vi "HFRR ADV v043.vi"() -> ()   [LabVIEW 2025] (continued)
  }
  n1338 = while {
    tunnel: w42 -> [_]
    tunnel: w28 -> [_]
    stop <- w1527 stop-if-true
    # "New Adv Logics"
    n1339 = local read "Main Tab"() -> (w1508:T2)
    n1340 = local read "Main Tab"() -> (w1525:T2)
    n1341 = local read "Sign In"() -> (w1524:bool)
    n1342 = case shown="\"Adv Scar\"" w1508 {
      frame "HOME", Default {
        n1343 = local read "LIVE FEED MIN TEMP"() -> (w1660:bool)
        n1344 = local write "LIVE FEED MAX TEMP"(TRUE ("LIVE FEED MAX TEMP")) -> ()
        n1345 = local read "CAMERA ROI MIN TEMP"() -> (w1658:bool)
        n1346 = case shown="True" w1660 {
          selector: w1660 -> [_ w1667]
          frame False {
          }
          frame True {
            n1347 = Not(x=w1667) -> (.not. x?=w1666:bool)
            n1348 = local write "LIVE FEED MIN TEMP"(w1666) -> ()
            n1349 = call "CAMERA LIVE FEED FGV.vi"("Enum - Menu"=CAMERA_LIVE_FEED_ENUM."CAMERA MINIMIZE") -> ()  [unwired: 9 in, 2 out]
          }
        }
        n1350 = case shown="True" w1658 {
          selector: w1658 -> [_ w1664]
          frame False {
          }
          frame True {
            n1351 = Not(x=w1664) -> (.not. x?=w1663:bool)
            n1352 = local write "CAMERA ROI MIN TEMP"(w1663) -> ()
            n1353 = call "IMAGE ANALYSIS.vi"("Enum"=POST_ANALYSIS_ENUM."MINIMIZE UI") -> ()  [unwired: 9 in, 2 out]
          }
        }
        n1354 = local write "CAMERA ROI MAX TEMP"(TRUE ("CAMERA ROI MAX TEMP")) -> ()
      }
      frame "Test Setup" {
        n1355 = local read "LIVE FEED MIN TEMP"() -> (w1670:bool)
        n1356 = local read "CAMERA ROI MIN TEMP"() -> (w1668:bool)
        n1357 = local write "LIVE FEED MAX TEMP"(TRUE ("LIVE FEED MAX TEMP")) -> ()
        n1358 = case shown="True" w1670 {
          selector: w1670 -> [_ w1677]
          frame False {
          }
          frame True {
            n1359 = Not(x=w1677) -> (.not. x?=w1676:bool)
            n1360 = local write "LIVE FEED MIN TEMP"(w1676) -> ()
            n1361 = call "CAMERA LIVE FEED FGV.vi"("Enum - Menu"=CAMERA_LIVE_FEED_ENUM."CAMERA MINIMIZE") -> ()  [unwired: 9 in, 2 out]
          }
        }
        n1362 = case shown="True" w1668 {
          selector: w1668 -> [_ w1674]
          frame False {
          }
          frame True {
            n1363 = Not(x=w1674) -> (.not. x?=w1673:bool)
            n1364 = local write "CAMERA ROI MIN TEMP"(w1673) -> ()
            n1365 = call "IMAGE ANALYSIS.vi"("Enum"=POST_ANALYSIS_ENUM."MINIMIZE UI") -> ()  [unwired: 9 in, 2 out]
          }
        }
        n1366 = local write "CAMERA ROI MAX TEMP"(TRUE ("CAMERA ROI MAX TEMP")) -> ()
      }
      frame "Acquire" {
        n1367 = local read "LIVE FEED MIN TEMP"() -> (w1680:bool)
        n1368 = local write "LIVE FEED MAX TEMP"(TRUE ("LIVE FEED MAX TEMP")) -> ()
        n1369 = local read "CAMERA ROI MIN TEMP"() -> (w1678:bool)
        n1370 = case shown="True" w1680 {
          selector: w1680 -> [_ w1687]
          frame False {
          }
          frame True {
            n1371 = Not(x=w1687) -> (.not. x?=w1686:bool)
            n1372 = local write "LIVE FEED MIN TEMP"(w1686) -> ()
            n1373 = call "CAMERA LIVE FEED FGV.vi"("Enum - Menu"=CAMERA_LIVE_FEED_ENUM."CAMERA MINIMIZE") -> ()  [unwired: 9 in, 2 out]
          }
        }
        n1374 = case shown="True" w1678 {
          selector: w1678 -> [_ w1684]
          frame False {
          }
          frame True {
            n1375 = Not(x=w1684) -> (.not. x?=w1683:bool)
            n1376 = local write "CAMERA ROI MIN TEMP"(w1683) -> ()
            n1377 = call "IMAGE ANALYSIS.vi"("Enum"=POST_ANALYSIS_ENUM."MINIMIZE UI") -> ()  [unwired: 9 in, 2 out]
          }
        }
        n1378 = local write "CAMERA ROI MAX TEMP"(TRUE ("CAMERA ROI MAX TEMP")) -> ()
      }
      frame "Adv Scar" {
        n1379 = local read "CAMERA ROI MIN TEMP"() -> (w1688:bool)
        n1380 = case shown="True" "LIVE FEED MAX TEMP" {
          selector: "LIVE FEED MAX TEMP" -> [_ w1709]
          frame False {
          }
          frame True {
            n1381 = Not(x=w1709) -> (.not. x?=w1708:bool)
            n1382 = local write "LIVE FEED MAX TEMP"(w1708) -> ()
            n1383 = call "CAMERA LIVE FEED FGV.vi"("Enum - Menu"=CAMERA_LIVE_FEED_ENUM."CAMERA RESTORE") -> ("error out"=w1699:errorcluster)  [unwired: 9 in, 1 out]
            n1384 = Type Cast(type=30, x=0) -> (*(type *) &x=w1703:i32)
            n1385 = Add(x=w1703, y=48) -> (x+y=w1704:i32)
            n1386 = call "CAMERA LIVE FEED FGV.vi"("Enum - Menu"=CAMERA_LIVE_FEED_ENUM."CAMERA MODE SET", "error in (no error)"=w1699, "CAMERA MODE"=w1704) -> ("error out"=w1696:errorcluster)  [unwired: 7 in, 1 out]
            n1387 = call "CAMERA LIVE FEED FGV.vi"("Enum - Menu"=CAMERA_LIVE_FEED_ENUM."CAMERA GRAY", "error in (no error)"=w1696) -> ("error out"=w1695:errorcluster)  [unwired: 8 in, 1 out]
            n1388 = call "LIST FILE NAMES.vi"("error in (no error)"=w1695) -> ("error out"=w1705:errorcluster, "filenames"=w1706:string[])  [unwired: 9 in]
            n1389 = property on="FILE 3" class="CmbBox"(error in=w1705, "Strings[]"=w1706) -> ()  [unwired: 1 in, 2 out]
          }
        }
        n1390 = case shown="True" w1688 {
          selector: w1688 -> [_ w1694]
          frame False {
          }
          frame True {
            n1391 = Not(x=w1694) -> (.not. x?=w1693:bool)
            n1392 = local write "CAMERA ROI MIN TEMP"(w1693) -> ()
            n1393 = call "IMAGE ANALYSIS.vi"("Enum"=POST_ANALYSIS_ENUM."MINIMIZE UI") -> ()  [unwired: 9 in, 2 out]
          }
        }
        n1394 = local write "CAMERA ROI MAX TEMP"(TRUE ("CAMERA ROI MAX TEMP")) -> ()
        "LIVE FEED MIN TEMP" <- TRUE ("LIVE FEED MIN TEMP")
      }
      frame "Adv Scar Report" {
        n1395 = local read "CAMERA ROI MAX TEMP"() -> (w1710:bool)
        n1396 = local read "LIVE FEED MIN TEMP"() -> (w1712:bool)
        n1397 = local write "LIVE FEED MAX TEMP"(TRUE ("LIVE FEED MAX TEMP")) -> ()
        n1398 = case shown="True" w1712 {
          selector: w1712 -> [_ w1721]
          frame False {
          }
          frame True {
            n1399 = Not(x=w1721) -> (.not. x?=w1720:bool)
            n1400 = local write "LIVE FEED MIN TEMP"(w1720) -> ()
            n1401 = call "CAMERA LIVE FEED FGV.vi"("Enum - Menu"=CAMERA_LIVE_FEED_ENUM."CAMERA MINIMIZE") -> ()  [unwired: 9 in, 2 out]
          }
        }
        n1402 = case shown="True" w1710 {
          selector: w1710 -> [_ w1718]
          frame False {
          }
          frame True {
            n1403 = Not(x=w1718) -> (.not. x?=w1716:bool)
            n1404 = local write "CAMERA ROI MAX TEMP"(w1716) -> ()
            n1405 = call "IMAGE ANALYSIS.vi"("Enum"=POST_ANALYSIS_ENUM."SHOW UI") -> ("error out"=w1715:errorcluster)  [unwired: 9 in, 1 out]
            n1406 = call "LIST FILE NAMES.vi"("error in (no error)"=w1715) -> ("filenames"=w1714:string[])  [unwired: 9 in, 1 out]
            n1407 = property on="Test File List :" class="CmbBox"("Strings[]"=w1714) -> ()  [unwired: 2 in, 2 out]
          }
        }
        n1408 = local write "CAMERA ROI MIN TEMP"(TRUE ("CAMERA ROI MIN TEMP")) -> ()
      }
      frame "Compare Files" {
        n1409 = local read "LIVE FEED MIN TEMP"() -> (w1724:bool)
        n1410 = local write "LIVE FEED MAX TEMP"(TRUE ("LIVE FEED MAX TEMP")) -> ()
        n1411 = local read "CAMERA ROI MIN TEMP"() -> (w1722:bool)
        n1412 = case shown="True" w1724 {
          selector: w1724 -> [_ w1731]
          frame False {
          }
          frame True {
            n1413 = Not(x=w1731) -> (.not. x?=w1730:bool)
            n1414 = local write "LIVE FEED MIN TEMP"(w1730) -> ()
            n1415 = call "CAMERA LIVE FEED FGV.vi"("Enum - Menu"=CAMERA_LIVE_FEED_ENUM."CAMERA MINIMIZE") -> ()  [unwired: 9 in, 2 out]
          }
        }
        n1416 = case shown="True" w1722 {
          selector: w1722 -> [_ w1728]
          frame False {
          }
          frame True {
            n1417 = Not(x=w1728) -> (.not. x?=w1727:bool)
            n1418 = local write "CAMERA ROI MIN TEMP"(w1727) -> ()
            n1419 = call "IMAGE ANALYSIS.vi"("Enum"=POST_ANALYSIS_ENUM."MINIMIZE UI") -> ()  [unwired: 9 in, 2 out]
          }
        }
        n1420 = local write "CAMERA ROI MAX TEMP"(TRUE ("CAMERA ROI MAX TEMP")) -> ()
      }
      frame "About" {
        n1421 = local read "LIVE FEED MIN TEMP"() -> (w1734:bool)
        n1422 = local write "LIVE FEED MAX TEMP"(TRUE ("LIVE FEED MAX TEMP")) -> ()
        n1423 = local read "CAMERA ROI MIN TEMP"() -> (w1733:bool)
        n1424 = case shown="True" w1734 {
          selector: w1734 -> [_ w1741]
          frame False {
          }
          frame True {
            n1425 = Not(x=w1741) -> (.not. x?=w1740:bool)
            n1426 = local write "LIVE FEED MIN TEMP"(w1740) -> ()
            n1427 = call "CAMERA LIVE FEED FGV.vi"("Enum - Menu"=CAMERA_LIVE_FEED_ENUM."CAMERA MINIMIZE") -> ()  [unwired: 9 in, 2 out]
          }
        }
        n1428 = case shown="True" w1733 {
          selector: w1733 -> [_ w1738]
          frame False {
          }
          frame True {
            n1429 = Not(x=w1738) -> (.not. x?=w1737:bool)
            n1430 = local write "CAMERA ROI MIN TEMP"(w1737) -> ()
            n1431 = call "IMAGE ANALYSIS.vi"("Enum"=POST_ANALYSIS_ENUM."MINIMIZE UI") -> ()  [unwired: 9 in, 2 out]
          }
        }
        n1432 = local write "CAMERA ROI MAX TEMP"(TRUE ("CAMERA ROI MIN TEMP")) -> ()
      }
      frame "Advance" {
        n1433 = local read "LIVE FEED MIN TEMP"() -> (w1744:bool)
        n1434 = local write "LIVE FEED MAX TEMP"(TRUE ("LIVE FEED MAX TEMP")) -> ()
        n1435 = local read "CAMERA ROI MIN TEMP"() -> (w1742:bool)
        n1436 = case shown="True" w1744 {
          selector: w1744 -> [_ w1751]
          frame False {
          }
          frame True {
            n1437 = Not(x=w1751) -> (.not. x?=w1750:bool)
            n1438 = local write "LIVE FEED MIN TEMP"(w1750) -> ()
            n1439 = call "CAMERA LIVE FEED FGV.vi"("Enum - Menu"=CAMERA_LIVE_FEED_ENUM."CAMERA MINIMIZE") -> ()  [unwired: 9 in, 2 out]
          }
        }
        n1440 = local write "CAMERA ROI MAX TEMP"(TRUE ("CAMERA ROI MAX TEMP")) -> ()
        n1441 = case shown="True" w1742 {
          selector: w1742 -> [_ w1748]
          frame False {
          }
          frame True {
            n1442 = Not(x=w1748) -> (.not. x?=w1747:bool)
            n1443 = local write "CAMERA ROI MIN TEMP"(w1747) -> ()
            n1444 = call "IMAGE ANALYSIS.vi"("Enum"=POST_ANALYSIS_ENUM."MINIMIZE UI") -> ()  [unwired: 9 in, 2 out]
          }
        }
      }
      frame "Mooha" {
        n1445 = local read "LIVE FEED MIN TEMP"() -> (w1754:bool)
        n1446 = local write "LIVE FEED MAX TEMP"(TRUE ("LIVE FEED MAX TEMP")) -> ()
        n1447 = local read "CAMERA ROI MIN TEMP"() -> (w1752:bool)
        n1448 = case shown="True" w1754 {
          selector: w1754 -> [_ w1761]
          frame False {
          }
          frame True {
            n1449 = Not(x=w1761) -> (.not. x?=w1760:bool)
            n1450 = local write "LIVE FEED MIN TEMP"(w1760) -> ()
            n1451 = call "CAMERA LIVE FEED FGV.vi"("Enum - Menu"=CAMERA_LIVE_FEED_ENUM."CAMERA MINIMIZE") -> ()  [unwired: 9 in, 2 out]
          }
        }
        n1452 = local write "CAMERA ROI MAX TEMP"(TRUE ("CAMERA ROI MAX TEMP")) -> ()
        n1453 = case shown="True" w1752 {
          selector: w1752 -> [_ w1758]
          frame False {
          }
          frame True {
            n1454 = Not(x=w1758) -> (.not. x?=w1757:bool)
            n1455 = local write "CAMERA ROI MIN TEMP"(w1757) -> ()
            n1456 = call "IMAGE ANALYSIS.vi"("Enum"=POST_ANALYSIS_ENUM."MINIMIZE UI") -> ()  [unwired: 9 in, 2 out]
          }
        }
      }
    }
    n1457 = local read "Auto Start Test"() -> (w1499:bool)
    n1458 = case shown="True" "sign in temp" {
      frame False {
      }
      frame True {
        w1534 = 1 ("y")
        n1459 = local read "USERNAME"() -> (w1540:string)
        n1460 = local read "USER ID"() -> (w1537:string)
        n1461 = call <vilib>:"Trim Whitespace.vi"("string"=w1540) -> ("trimmed string"=w1539:string)  [unwired: 1 in]
        n1462 = call <vilib>:"Trim Whitespace.vi"("string"=w1537) -> ("trimmed string"=w1538:string)  [unwired: 1 in]
        n1463 = String Length(string=w1539) -> (length=w1536:i32)
        n1464 = String Length(string=w1538) -> (length=w1535:i32)
        n1465 = Greater?(x=w1536, y=w1534) -> (0:w1533:bool)
        n1466 = Greater?(x=w1535, y=w1534) -> (0:w1532:bool)
        n1467 = And(x=w1533, y=w1532) -> (x .and. y?=w1531:bool)
        n1468 = case shown="True" w1531 {
          frame False {
            n1469 = property on="Sign In" class="Bool (strict)"("DisabledEnum"=T19."Disabled" ("Disabled")) -> ()  [unwired: 2 in, 2 out]
          }
          frame True {
            n1470 = property on="Sign In" class="Bool (strict)"("DisabledEnum"=T19."Enabled" ("Disabled")) -> ()  [unwired: 2 in, 2 out]
          }
        }
      }
    }
    n1471 = local read "Air Temperature"() -> (w1516:bool)
    n1472 = local read "Coefficient Of Friction"() -> (w1517:bool)
    n1473 = case shown="False" w1499 {
      frame False {
        n1474 = local read "Auto stop temp"() -> (w1528:bool)
        n1475 = case shown="True" w1528 {
          frame False {
          }
          frame True {
            n1476 = local write "Auto Start Temp"(FALSE ("Auto Start Temp")) -> ()
          }
        }
      }
      frame True {
        "Auto stop temp" <- TRUE ("Auto stop temp")
      }
    }
    n1477 = local read "Humidity 3"() -> (w1515:bool)
    n1478 = case shown="\"HOME\"" w1525 {
      frame "HOME" {
        n1479 = local write "main tab sub"(enum32{"Page 1", "Page 2"}."Page 1" ("main tab sub")) -> ()
      }
      frame Default {
        n1480 = local write "main tab sub"(enum32{"Page 1", "Page 2"}."Page 2" ("main tab sub")) -> ()
      }
    }
    n1481 = case shown="True" w1524 {
      selector: w1524 -> [_ w1876]
      frame False {
      }
      frame True {
        n1482 = Not(x=w1876) -> (.not. x?=w1875:bool)
        n1483 = local write "Sign In"(w1875) -> ()
        n1484 = local write "Main Dashboard Buttons"(T25."Test Setup" ("Main Dashboard Buttons")) -> ()
      }
    }
    n1485 = case shown="\"Numeric Display\", Default" "Num/Graph" {
      frame "Numeric Display", Default {
        n1486 = property on="Single/Multiple" class="RadioBtnsControl (strict)"("Visible"=FALSE) -> ()  [unwired: 2 in, 2 out]
        n1487 = property on="Single - Graph" class="Ring (strict)"("Visible"=FALSE) -> ()  [unwired: 2 in, 2 out]
        n1488 = local write "Main Tab Display"(T4."Dashboard 1" ("Main Tab Display")) -> ()
      }
      frame "Graph Display" {
        n1489 = property on="Single/Multiple" class="RadioBtnsControl (strict)"("Visible"=TRUE) -> ()  [unwired: 2 in, 2 out]
        n1490 = case shown="\"Multiple\"" "Single/Multiple" {
          frame "Single ", Default {
            n1491 = property on="Single - Graph" class="Ring (strict)"("Visible"=TRUE) -> ()  [unwired: 2 in, 2 out]
            n1492 = local write "Main Tab Display"(T4."Dashboard 3" ("Main Tab Display")) -> ()
          }
          frame "Multiple" {
            n1493 = property on="Single - Graph" class="Ring (strict)"("Visible"=FALSE) -> ()  [unwired: 2 in, 2 out]
            n1494 = local write "Main Tab Display"(T4."Dashboard 2" ("Main Tab Display")) -> ()
          }
        }
      }
    }
    n1495 = local read "Stroke"() -> (w1514:bool)
    n1496 = local read "USERNAME"() -> (w1519:string)
    n1497 = case shown="True" w1517 {
      selector: w1517 -> [_ w1801]
      frame False {
      }
      frame True {
        n1498 = Not(x=w1801) -> (.not. x?=w1800:bool)
        n1499 = local write "Coefficient Of Friction"(w1800) -> ()
        n1500 = local write "Tab Control 2"(T6."Coefficient Of Friction" ("Tab Control 2")) -> ()
      }
    }
    n1501 = case shown="True" w1516 {
      selector: w1516 -> [_ w1798]
      frame False {
      }
      frame True {
        n1502 = Not(x=w1798) -> (.not. x?=w1796:bool)
        n1503 = local write "Air Temperature"(w1796) -> ()
        n1504 = local write "Tab Control 2"(T6."Air Temperature" ("Tab Control 2")) -> ()
      }
    }
    n1505 = case shown="True" w1514 {
      selector: w1514 -> [_ w1792]
      frame False {
      }
      frame True {
        n1506 = Not(x=w1792) -> (.not. x?=w1790:bool)
        n1507 = local write "Stroke"(w1790) -> ()
        n1508 = local write "Tab Control 2"(T6."Stroke" ("Tab Control 2")) -> ()
      }
    }
    n1509 = local write "tested by"(w1519) -> ()
    n1510 = case shown="True" w1515 {
      selector: w1515 -> [_ w1795]
      frame False {
      }
      frame True {
        n1511 = Not(x=w1795) -> (.not. x?=w1793:bool)
        n1512 = local write "Humidity 3"(w1793) -> ()
        n1513 = local write "Tab Control 2"(T6."Humidity" ("Tab Control 2")) -> ()
      }
    }
    n1514 = case shown="\"Calibration\"" "Main Dashboard Buttons" {
      tunnel: [T2."HOME" ("Main Tab") T2."Test Setup" ("Main Tab") T2."Acquire" ("Main Tab") T2."Adv Scar" ("Main Tab") T2."Adv Scar Report" ("Main Tab") T2."Compare Files" ("Main Tab") T2."Calibration" ("Main Tab") T2."About" ("Main Tab") T2."Advance" ("Main Tab")] -> w1498
      frame "Home", Default {
      }
      frame "Test Setup" {
      }
      frame "Dashboard" {
      }
      frame "Imaging" {
      }
      frame "Report" {
      }
      frame "Analysis" {
      }
      frame "Calibration" {
      }
      frame "About" {
      }
      frame "Advance" {
      }
    }
    n1515 = Wait (ms)(milliseconds to wait=u32 100) -> ()  [unwired: 1 out]
    n1516 = local read "Main Tab Display"() -> (w1518:T4)
    n1517 = local write "Main Tab"(w1498) -> ()
    n1518 = case shown="\"Dashboard 3\"" w1518 {
      frame "Dashboard 1", Default {
        n1519 = property on="Reset Graph" class="Bool (strict)"("Visible"=FALSE) -> ()  [unwired: 2 in, 2 out]
      }
      frame "Dashboard 2" {
        n1520 = property on="Reset Graph" class="Bool (strict)"("Visible"=TRUE) -> ()  [unwired: 2 in, 2 out]
      }
      frame "Dashboard 3" {
        n1521 = property on="Reset Graph" class="Bool (strict)"("Visible"=TRUE) -> ()  [unwired: 2 in, 2 out]
      }
    }
    n1522 = local read "SCAR MEASURMENT"() -> (w1506:enum32{"Auto Scar", "Manual Scar"})
    n1523 = local read "Humidity"() -> (w1520:bool)
    n1524 = local read "Cap Live Image"() -> (w1503:bool)
    n1525 = local read "Sample Temperature"() -> (w1513:bool)
    n1526 = local read "Air Temp vs Humidity"() -> (w1511:bool)
    n1527 = local read "Frequency"() -> (w1512:bool)
    n1528 = case shown="False" w1520 {
      frame False {
        n1529 = local write "Humidity On Command"(TRUE ("Humidity On Command")) -> ()
        n1530 = case shown="True" "Humidity Off Command" {
          selector: "Humidity Off Command" -> [_ w1808]
          frame False {
          }
          frame True {
            n1531 = stacked-sequence {
              frame #0 {
                n1532 = local read "WriteHumidity"() -> (w1810:string[])
                n1533 = Insert Into Array(array=w1810, new element="R;1" ("new element/subarray")) -> (w1809:string[])  [unwired: 1 in]
                n1534 = local write "WriteHumidity"(w1809) -> ()
              }
              frame #1 {
                n1535 = Wait (ms)(milliseconds to wait=u32 500) -> ()  [unwired: 1 out]
              }
              frame #2 {
                n1536 = local read "WriteHumidity"() -> (w1814:string[])
                n1537 = local read "EVENT LOG"() -> (w1818:string)
                n1538 = call "Event Log.vi"("Content"="Humidity Control Off" ("string"), "EVENT LOG"=w1818) -> ("EVENT LOG"=w1819:string)  [unwired: 8 in, 1 out]
                n1539 = local write "EVENT LOG"(w1819) -> ()
                n1540 = Insert Into Array(array=w1814, new element="R;1" ("new element/subarray")) -> (w1815:string[])  [unwired: 1 in]
                n1541 = local write "WriteHumidity"(w1815) -> ()
                n1542 = local write "Humidity 2"(TRUE ("Humidity")) -> ()
              }
            }
            n1543 = Not(x=w1808) -> (.not. x?=w1807:bool)
            n1544 = local write "Humidity Off Command"(w1807) -> ()
          }
        }
      }
      frame True {
        n1545 = local write "Humidity Off Command"(TRUE ("Humidity Off Command")) -> ()
        n1546 = case shown="False" "Humidity On Command" {
          selector: "Humidity On Command" -> [_ w1823]
          frame False {
          }
          frame True {
            n1547 = stacked-sequence {
              frame #0 {
                n1548 = local read "Set Rh"() -> (w1829:dbl)
                n1549 = local read "WriteHumidity"() -> (w1825:string[])
                n1550 = Number To Fractional String(number=w1829, precision (6)=i16 2) -> (F-format string=w1830:string)  [unwired: 2 in]
                n1551 = Concatenate Strings("M;" ("new element/subarray"), w1830) -> (w1828:string)
                n1552 = Insert Into Array(array=w1825, new element=w1828) -> (w1824:string[])  [unwired: 1 in]
                n1553 = local write "WriteHumidity"(w1824) -> ()
              }
              frame #1 {
                n1554 = Wait (ms)(milliseconds to wait=u32 500) -> ()  [unwired: 1 out]
              }
              frame #2 {
                n1555 = local read "WriteHumidity"() -> (w1833:string[])
                n1556 = local read "Set Rh"() -> (w1837:dbl)
                n1557 = Number To Fractional String(number=w1837, precision (6)=i16 2) -> (F-format string=w1838:string)  [unwired: 2 in]
                n1558 = Concatenate Strings("M;" ("new element/subarray"), w1838) -> (w1836:string)
                n1559 = Insert Into Array(array=w1833, new element=w1836) -> (w1832:string[])  [unwired: 1 in]
                n1560 = local write "WriteHumidity"(w1832) -> ()
              }
              frame #3 {
                n1561 = Wait (ms)(milliseconds to wait=u32 500) -> ()  [unwired: 1 out]
              }
              frame #4 {
                (unwired) "% RH" ("string")
                (unwired) i16 2 ("precision (6)")
                (unwired) "M;" ("new element/subarray")
                n1562 = local read "Set Rh"() -> (w1847:dbl)
                n1563 = local read "WriteHumidity"() -> (w1840:string[])
                n1564 = Number To Fractional String(number=w1847, precision (6)=i16 2) -> (F-format string=w1844:string)  [unwired: 2 in]
                n1565 = Concatenate Strings("M;" ("new element/subarray"), w1844) -> (w1848:string)
                n1566 = Concatenate Strings("Humidity Set to : " ("string"), w1844, "% RH" ("string")) -> (w1842:string)
                n1567 = Insert Into Array(array=w1840, new element=w1848) -> (w1841:string[])  [unwired: 1 in]
                n1568 = disable-structure shown="Enabled" {
                  frame Enabled {
                    n1569 = local read "EVENT LOG"() -> (w1851:string)
                    n1570 = call "Event Log.vi"("Content"="Humidity Control On", "EVENT LOG"=w1851) -> ("EVENT LOG"=w1852:string)  [unwired: 8 in, 1 out]
                    n1571 = local write "EVENT LOG"(w1852) -> ()
                  }
                  frame Disabled {
                  }
                }
                n1572 = disable-structure shown="Enabled" {
                  disable-tunnel: w1842 -> [_ _]
                  frame Enabled {
                    n1573 = local read "EVENT LOG"() -> (w1854:string)
                    n1574 = call "Event Log.vi"("Content"="Humidity Control On", "EVENT LOG"=w1854) -> ("EVENT LOG"=w1855:string)  [unwired: 8 in, 1 out]
                    n1575 = local write "EVENT LOG"(w1855) -> ()
                  }
                  frame Disabled {
                  }
                }
                n1576 = local write "WriteHumidity"(w1841) -> ()
              }
            }
            n1577 = Not(x=w1823) -> (.not. x?=w1822:bool)
            n1578 = local write "Humidity On Command"(w1822) -> ()
          }
        }
      }
    }
    n1579 = Equal?(x=w1506, y=enum32{"Auto Scar", "Manual Scar"}."Auto Scar" ("SCAR MEASURMENT")) -> (x = y?=w1502:bool)
    n1580 = local read "TEST STANDARD"() -> (w1509:T3)
    n1581 = And(x=w1503, y=w1502) -> (x .and. y?=w1504:bool)
    n1582 = case shown="True" w1504 {
      selector: w1504 -> [_ w1607]
      tunnel: errorcluster {"status"=FALSE, "code"=0, "source"=""} ("error in (no error) 3") -> [_ w1608]
      frame False {
      }
      frame True {
        n1583 = stacked-sequence {
          tunnel: w1608 -> [_ _ _ _ _ _ _ w1656]
          tunnel: w1607 -> [_ _ _ _ _ w1637 _ _]
          frame #0 {
            n1584 = call "CAMERA LIVE FEED FGV.vi"("Enum - Menu"=CAMERA_LIVE_FEED_ENUM."CAMERA MINIMIZE") -> ()  [unwired: 9 in, 2 out]
          }
          frame #1 {
            n1585 = property on="Auto Scar Check  2" class="Clust (strict)"("Visible"=TRUE) -> ()  [unwired: 2 in, 2 out]
          }
          frame #2 {
            n1586 = String To Path(string="C:\\LAB-IQ\\Image Calibrate v01.dcf") -> (path=w1613:path)
            n1587 = Open/Create/Replace File ("Open File")(file path (use dialog)=w1613) -> (refnum out=w1614:refnum<file>)  [unwired: 5 in, 2 out]
            n1588 = for {
              N: 4 -> [_]
              tunnel: w1614 -> [w1620]
              i -> [w1616]
              n1589 = Read from Text File ("Read File")(file (use dialog)=w1620) -> (text=w1621:string)  [unwired: 3 in, 3 out]
              n1590 = String Subset(string=w1621, offset (0)=6, length (rest)=10 ("length (rest)")) -> (substring=w1617:string)
              n1591 = Fract/Exp String To Number(string=w1617) -> (number=w1615:dbl)  [unwired: 3 in, 1 out]
              n1592 = case shown="0" w1616 {
                tunnel: w1615 -> [w1622 w1623 _ w1624 _]
                frame 0 {
                  "5x Gain" <- w1622
                }
                frame 1 {
                  "10x Gain" <- w1623
                }
                frame 2 {
                }
                frame 3 {
                  "100x gain" <- w1624
                }
                frame 4, Default {
                }
              }
            }
          }
          frame #3 {
            n1593 = local read "FILE 3"() -> (w1630:string)
            n1594 = call <vilib>:"Trim Whitespace.vi"("string"="C:\\LAB-IQ\\images\\") -> ("trimmed string"=w1632:string)  [unwired: 1 in]
            n1595 = String To Path(string=w1632) -> (path=w1631:path)
            n1596 = Concatenate Strings(w1630, ".png" ("string")) -> (w1629:string)
            n1597 = Build Path(base path=w1631, name or relative path=w1629) -> (appended path=w1627:path)
            "Image path" <- w1627
            n1598 = Path To String(path=w1627) -> (string=w1626:string)
            n1599 = call "CAMERA LIVE FEED FGV.vi"("Enum - Menu"=CAMERA_LIVE_FEED_ENUM."CAMERA SAVE", "Image Path"=w1626) -> ()  [unwired: 8 in, 2 out]
          }
          frame #4 {
            n1600 = One Button Dialog(message="Image saved successfully") -> ()  [unwired: 1 in, 1 out]
          }
          frame #5 {
            n1601 = local read "TEST STANDARD"() -> (w1636:T3)
            n1602 = local read "Magnification len live scar"() -> (w1648:string)
            n1603 = Not(x=w1637) -> (.not. x?=w1638:bool)
            n1604 = local write "Cap Live Image"(w1638) -> ()
            n1605 = case shown="\"ISO 12156\"" w1636 {
              tunnel: ["ASTM D6079" "ISO 12156"] -> w1635
              frame "ASTM D6079", Default {
              }
              frame "ISO 12156" {
              }
            }
            n1606 = case shown="\"5x\", Default" w1648 {
              tunnel: [w1651 w1652] -> w1647
              frame "5x", Default {
                n1607 = local read "5x Gain"() -> (w1651:dbl)
              }
              frame "10x" {
                # "5x"
                n1608 = local read "10x Gain"() -> (w1652:dbl)
              }
            }
            n1609 = local read "Image path"() -> (w1646:path)
            n1610 = local read "FILE 3"() -> (w1639:string)
            n1611 = call "EDGE DETCTION.vi"("GAIN VALUE"=w1647, "Image Path"=w1646) -> ("error out"=w1645:errorcluster, "return value"=w1644:cluster{string, string, dbl, dbl, dbl})  [unwired: 8 in]
            n1612 = Bundle By Name(cluster=T26 {"File Name"="", "Test Method"="", "Operator"="", "Fuel Description"="", "Date and time"=""} ("Main Ref"), "File Name"=w1639, "Test Method"=w1635) -> (w1640:T26)
            n1613 = call "duf file read.vi"("error in (no error)"=w1645, "Main Ref"=w1640) -> ("error out"=w1643:errorcluster, "Main Ref 2"=w1641:T26)  [unwired: 8 in]
            n1614 = call "EDGE DETECTION REPORT.vi"("error in (no error)"=w1643, "return value 2"=w1644, "Main Ref"=w1641) -> ()  [unwired: 8 in, 1 out]
          }
          frame #6 {
            n1615 = property on="Auto Scar Check  2" class="Clust (strict)"("Visible"=FALSE) -> ()  [unwired: 2 in, 2 out]
          }
          frame #7 {
            n1616 = call "CAMERA LIVE FEED FGV.vi"("Enum - Menu"=CAMERA_LIVE_FEED_ENUM."CAMERA MINIMIZE", "error in (no error)"=w1656) -> ()  [unwired: 8 in, 2 out]
            n1617 = local write "Main Dashboard Buttons"(T1."Home" ("Main Dashboard Buttons")) -> ()
            n1618 = local write "Main Tab"(T2."HOME" ("Main Tab")) -> ()
          }
        }
      }
    }
    n1619 = local read "Heater Button"() -> (w1510:bool)
    n1620 = case shown="True" w1512 {
      selector: w1512 -> [_ w1786]
      frame False {
      }
      frame True {
        n1621 = Not(x=w1786) -> (.not. x?=w1784:bool)
        n1622 = local write "Frequency"(w1784) -> ()
        n1623 = local write "Tab Control 2"(T6."Frequency" ("Tab Control 2")) -> ()
      }
    }
    n1624 = case shown="True" w1511 {
      selector: w1511 -> [_ w1783]
      frame False {
      }
      frame True {
        n1625 = Not(x=w1783) -> (.not. x?=w1781:bool)
        n1626 = local write "Air Temp vs Humidity"(w1781) -> ()
        n1627 = local write "Tab Control 2"(T6."Air Temp vs Rh" ("Tab Control 2")) -> ()
      }
    }
    n1628 = case shown="True" w1513 {
      selector: w1513 -> [_ w1789]
      frame False {
      }
      frame True {
        n1629 = Not(x=w1789) -> (.not. x?=w1787:bool)
        n1630 = local write "Sample Temperature"(w1787) -> ()
        n1631 = local write "Tab Control 2"(T6."Sample Temperature" ("Tab Control 2")) -> ()
      }
    }
    n1632 = case shown="\"Custom\"" w1509 {
      frame "ASTM D6079", Default {
        w1762 = "ASTM D6079 TEST CONDITIONS" ("Standard 2")
        n1633 = local write "Standard 2"(w1762) -> ()
        n1634 = local write "Standard"(w1762) -> ()
      }
      frame "ISO 12156" {
        w1763 = "ISO 12156 TEST CONDITIONS" ("Standard 2")
        n1635 = local write "Standard 2"(w1763) -> ()
        n1636 = local write "Standard"(w1763) -> ()
      }
      frame "CEC F-096-A-06" {
        w1764 = "CEC F-096-A-06 TEST CONDITIONS" ("Standard 2")
        n1637 = local write "Standard 2"(w1764) -> ()
        n1638 = local write "Standard"(w1764) -> ()
      }
      frame "Custom" {
        w1765 = "CUSTOM TEST CONDITIONS" ("Standard 2")
        n1639 = local write "Standard 2"(w1765) -> ()
        n1640 = local write "Standard"(w1765) -> ()
      }
    }
    n1641 = case shown="True" w1510 {
      frame False {
        n1642 = local write "Temperature On Command"(TRUE ("Temperature On Command")) -> ()
        n1643 = case shown="True" "Temperature Off Command" {
          selector: "Temperature Off Command" -> [_ w1769]
          frame False {
          }
          frame True {
            n1644 = Not(x=w1769) -> (.not. x?=w1768:bool)
            n1645 = local read "EVENT LOG"() -> (w1772:string)
            n1646 = local write "Temperature Off Command"(w1768) -> ()
            n1647 = call "Event Log.vi"("Content"="Heater Off", "EVENT LOG"=w1772) -> ("EVENT LOG"=w1771:string)  [unwired: 8 in, 1 out]
            n1648 = local write "EVENT LOG"(w1771) -> ()
          }
        }
      }
      frame True {
        n1649 = local write "Temperature Off Command"(TRUE ("Temperature Off Command")) -> ()
        n1650 = case shown="True" "Temperature On Command" {
          selector: "Temperature On Command" -> [_ w1776]
          frame False {
          }
          frame True {
            n1651 = Not(x=w1776) -> (.not. x?=w1775:bool)
            n1652 = local write "Temperature On Command"(w1775) -> ()
            n1653 = disable-structure shown="Enabled" {
              disable-tunnel: "Heater On" -> [w1778 _]
              frame Enabled {
                n1654 = local read "EVENT LOG"() -> (w1779:string)
                n1655 = call "Event Log.vi"("Content"=w1778, "EVENT LOG"=w1779) -> ("EVENT LOG"=w1780:string)  [unwired: 8 in, 1 out]
                n1656 = local write "EVENT LOG"(w1780) -> ()
              }
              frame Disabled {
              }
            }
          }
        }
      }
    }
    n1657 = local read "Main Tab"() -> (w1501:T2)
    n1658 = case shown="\"About\"" w1501 {
      frame "HOME", Default {
        w1543 = T19."Enabled" ("Disabled")
        n1659 = local read "Service Password enable"() -> (w1545:bool)
        n1660 = property on="Imaging" class="Bool (strict)"("DisabledEnum"=w1543) -> ()  [unwired: 2 in, 2 out]
        n1661 = property on="Dashboard" class="Bool (strict)"("DisabledEnum"=w1543) -> ()  [unwired: 2 in, 2 out]
        n1662 = property on="Test Setup" class="Bool (strict)"("DisabledEnum"=w1543) -> ()  [unwired: 2 in, 2 out]
        n1663 = property on="Analysis" class="Bool (strict)"("DisabledEnum"=w1543) -> ()  [unwired: 2 in, 2 out]
        n1664 = property on="Home" class="Bool (strict)"("DisabledEnum"=w1543) -> ()  [unwired: 2 in, 2 out]
        n1665 = property on="Report" class="Bool (strict)"("DisabledEnum"=w1543) -> ()  [unwired: 2 in, 2 out]
        n1666 = property on="Main Dashboard Buttons" class="RadioBtnsControl (strict)"("DisabledEnum"=w1543) -> ()  [unwired: 2 in, 2 out]
        n1667 = property on="Calibration" class="Bool (strict)"("DisabledEnum"=w1543) -> ()  [unwired: 2 in, 2 out]
        n1668 = case shown="True" w1545 {
          tunnel: [T19."Disabled" ("Disabled") T19."Enabled" ("Disabled")] -> w1544
          frame False {
          }
          frame True {
          }
        }
        n1669 = property on="About" class="Bool (strict)"("DisabledEnum"=w1544) -> ()  [unwired: 2 in, 2 out]
      }
      frame "Test Setup" {
        w1550 = T19."Enabled" ("Disabled")
        n1670 = local read "Service Password enable"() -> (w1549:bool)
        n1671 = property on="Dashboard" class="Bool (strict)"("DisabledEnum"=T19."Disabled" ("Disabled")) -> ()  [unwired: 2 in, 2 out]
        n1672 = property on="Imaging" class="Bool (strict)"("DisabledEnum"=w1550) -> ()  [unwired: 2 in, 2 out]
        n1673 = property on="Analysis" class="Bool (strict)"("DisabledEnum"=w1550) -> ()  [unwired: 2 in, 2 out]
        n1674 = property on="Home" class="Bool (strict)"("DisabledEnum"=w1550) -> ()  [unwired: 2 in, 2 out]
        n1675 = property on="Report" class="Bool (strict)"("DisabledEnum"=w1550) -> ()  [unwired: 2 in, 2 out]
        n1676 = property on="Test Setup" class="Bool (strict)"("DisabledEnum"=w1550) -> ()  [unwired: 2 in, 2 out]
        n1677 = case shown="True" w1549 {
          tunnel: [T19."Disabled" ("Disabled") T19."Enabled" ("Disabled")] -> w1548
          frame False {
          }
          frame True {
          }
        }
        n1678 = property on="About" class="Bool (strict)"("DisabledEnum"=w1548) -> ()  [unwired: 2 in, 2 out]
      }
      frame "Adv Scar" {
        w1557 = T19."Enabled" ("Disabled")
        n1679 = property on="Dashboard" class="Bool (strict)"("DisabledEnum"=T19."Disabled" ("Disabled")) -> ()  [unwired: 2 in, 2 out]
        n1680 = property on="Imaging" class="Bool (strict)"("DisabledEnum"=w1557) -> ()  [unwired: 2 in, 2 out]
        n1681 = property on="Analysis" class="Bool (strict)"("DisabledEnum"=w1557) -> ()  [unwired: 2 in, 2 out]
        n1682 = property on="Home" class="Bool (strict)"("DisabledEnum"=w1557) -> ()  [unwired: 2 in, 2 out]
        n1683 = property on="Report" class="Bool (strict)"("DisabledEnum"=w1557) -> ()  [unwired: 2 in, 2 out]
        n1684 = property on="Test Setup" class="Bool (strict)"("DisabledEnum"=w1557) -> ()  [unwired: 2 in, 2 out]
        n1685 = local read "Service Password enable"() -> (w1555:bool)
        n1686 = case shown="True" w1555 {
          tunnel: [T19."Disabled" ("Disabled") T19."Enabled" ("Disabled")] -> w1554
          frame False {
          }
          frame True {
          }
        }
        n1687 = property on="About" class="Bool (strict)"("DisabledEnum"=w1554) -> ()  [unwired: 2 in, 2 out]
      }
      frame "Calibration" {
        w1560 = T19."Enabled" ("Disabled")
        n1688 = property on="Dashboard" class="Bool (strict)"("DisabledEnum"=T19."Disabled" ("Disabled")) -> ()  [unwired: 2 in, 2 out]
        n1689 = property on="Imaging" class="Bool (strict)"("DisabledEnum"=w1560) -> ()  [unwired: 2 in, 2 out]
        n1690 = property on="Analysis" class="Bool (strict)"("DisabledEnum"=w1560) -> ()  [unwired: 2 in, 2 out]
        n1691 = property on="Home" class="Bool (strict)"("DisabledEnum"=w1560) -> ()  [unwired: 2 in, 2 out]
        n1692 = property on="Report" class="Bool (strict)"("DisabledEnum"=w1560) -> ()  [unwired: 2 in, 2 out]
        n1693 = property on="Test Setup" class="Bool (strict)"("DisabledEnum"=w1560) -> ()  [unwired: 2 in, 2 out]
        n1694 = local read "Service Password enable"() -> (w1562:bool)
        n1695 = property on="Calibration" class="Bool (strict)"("DisabledEnum"=w1560) -> ()  [unwired: 2 in, 2 out]
        n1696 = case shown="True" w1562 {
          tunnel: [T19."Disabled" ("Disabled") T19."Enabled" ("Disabled")] -> w1561
          frame False {
          }
          frame True {
          }
        }
        n1697 = property on="About" class="Bool (strict)"("DisabledEnum"=w1561) -> ()  [unwired: 2 in, 2 out]
      }
      frame "Adv Scar Report" {
        w1568 = T19."Enabled" ("Disabled")
        n1698 = property on="Dashboard" class="Bool (strict)"("DisabledEnum"=T19."Disabled" ("Disabled")) -> ()  [unwired: 2 in, 2 out]
        n1699 = property on="Imaging" class="Bool (strict)"("DisabledEnum"=w1568) -> ()  [unwired: 2 in, 2 out]
        n1700 = property on="Analysis" class="Bool (strict)"("DisabledEnum"=w1568) -> ()  [unwired: 2 in, 2 out]
        n1701 = property on="Home" class="Bool (strict)"("DisabledEnum"=w1568) -> ()  [unwired: 2 in, 2 out]
        n1702 = property on="Report" class="Bool (strict)"("DisabledEnum"=w1568) -> ()  [unwired: 2 in, 2 out]
        n1703 = property on="Test Setup" class="Bool (strict)"("DisabledEnum"=w1568) -> ()  [unwired: 2 in, 2 out]
        n1704 = local read "Service Password enable"() -> (w1567:bool)
        n1705 = case shown="True" w1567 {
          tunnel: [T19."Disabled" ("Disabled") T19."Enabled" ("Disabled")] -> w1566
          frame False {
          }
          frame True {
          }
        }
        n1706 = property on="About" class="Bool (strict)"("DisabledEnum"=w1566) -> ()  [unwired: 2 in, 2 out]
      }
      frame "Compare Files" {
        w1574 = T19."Enabled" ("Disabled")
        n1707 = local read "Service Password enable"() -> (w1573:bool)
        n1708 = property on="Dashboard" class="Bool (strict)"("DisabledEnum"=T19."Disabled" ("Disabled")) -> ()  [unwired: 2 in, 2 out]
        n1709 = property on="Imaging" class="Bool (strict)"("DisabledEnum"=w1574) -> ()  [unwired: 2 in, 2 out]
        n1710 = property on="Analysis" class="Bool (strict)"("DisabledEnum"=w1574) -> ()  [unwired: 2 in, 2 out]
        n1711 = property on="Home" class="Bool (strict)"("DisabledEnum"=w1574) -> ()  [unwired: 2 in, 2 out]
        n1712 = property on="Report" class="Bool (strict)"("DisabledEnum"=w1574) -> ()  [unwired: 2 in, 2 out]
        n1713 = property on="Test Setup" class="Bool (strict)"("DisabledEnum"=w1574) -> ()  [unwired: 2 in, 2 out]
        n1714 = case shown="True" w1573 {
          tunnel: [T19."Disabled" ("Disabled") T19."Enabled" ("Disabled")] -> w1572
          frame False {
          }
          frame True {
          }
        }
        n1715 = property on="About" class="Bool (strict)"("DisabledEnum"=w1572) -> ()  [unwired: 2 in, 2 out]
      }
      frame "Acquire" {
        n1716 = local read "Service Password enable"() -> (w1579:bool)
        n1717 = property on="Test Setup" class="Bool (strict)"("DisabledEnum"=T19."Disabled" ("Disabled")) -> ()  [unwired: 2 in, 2 out]
        n1718 = local read "Auto Start Test"() -> (w1581:bool)
        n1719 = local read "RUN"() -> (w1583:bool)
        n1720 = case shown="True" w1579 {
          tunnel: [T19."Disabled" ("Disabled") T19."Enabled" ("Disabled")] -> w1580
          frame False {
          }
          frame True {
          }
        }
        n1721 = Or(x=w1583, y=w1581) -> (x .or. y?=w1582:bool)
        n1722 = case shown="True" w1582 {
          tunnel: [T19."Enabled" ("Disabled") T19."Disabled" ("Disabled")] -> w1578
          frame False {
          }
          frame True {
          }
        }
        n1723 = property on="About" class="Bool (strict)"("DisabledEnum"=w1580) -> ()  [unwired: 2 in, 2 out]
        n1724 = property on="Imaging" class="Bool (strict)"("DisabledEnum"=w1578) -> ()  [unwired: 2 in, 2 out]
        n1725 = property on="Dashboard" class="Bool (strict)"("DisabledEnum"=w1578) -> ()  [unwired: 2 in, 2 out]
        n1726 = property on="Analysis" class="Bool (strict)"("DisabledEnum"=w1578) -> ()  [unwired: 2 in, 2 out]
        n1727 = property on="Home" class="Bool (strict)"("DisabledEnum"=w1578) -> ()  [unwired: 2 in, 2 out]
        n1728 = property on="Report" class="Bool (strict)"("DisabledEnum"=w1578) -> ()  [unwired: 2 in, 2 out]
        n1729 = property on="Calibration" class="Bool (strict)"("DisabledEnum"=w1578) -> ()  [unwired: 2 in, 2 out]
      }
      frame "About" {
        n1730 = local read "FILE"() -> (w1597:string)
        n1731 = local read "TEST FILE NAM,E SAVED"() -> (w1590:bool)
        n1732 = call <vilib>:"Trim Whitespace.vi"("string"=w1597) -> ("trimmed string"=w1596:string)  [unwired: 1 in]
        n1733 = local read "Auto Start Test"() -> (w1600:bool)
        n1734 = String Length(string=w1596) -> (length=w1595:i32)
        n1735 = Greater?(x=w1595, y=1) -> (0:w1592:bool)
        n1736 = And(x=w1592, y=w1590) -> (x .and. y?=w1591:bool)
        n1737 = local read "RUN"() -> (w1602:bool)
        n1738 = case shown="True" w1591 {
          tunnel: [T19."Disabled" ("Disabled") T19."Enabled" ("Disabled")] -> w1593
          frame False {
          }
          frame True {
          }
        }
        n1739 = Or(x=w1602, y=w1600) -> (x .or. y?=w1601:bool)
        n1740 = property on="About" class="Bool (strict)"("DisabledEnum"=T19."Enabled" ("Disabled")) -> ()  [unwired: 2 in, 2 out]
        n1741 = case shown="False" w1601 {
          tunnel: [T19."Enabled" ("Disabled") T19."Disabled" ("Disabled")] -> w1599
          frame False {
          }
          frame True {
          }
        }
        n1742 = property on="Dashboard" class="Bool (strict)"("DisabledEnum"=w1593) -> ()  [unwired: 2 in, 2 out]
        n1743 = property on="Test Setup" class="Bool (strict)"("DisabledEnum"=T19."Disabled" ("Disabled")) -> ()  [unwired: 2 in, 2 out]
        n1744 = property on="Imaging" class="Bool (strict)"("DisabledEnum"=w1599) -> ()  [unwired: 2 in, 2 out]
        n1745 = property on="Analysis" class="Bool (strict)"("DisabledEnum"=w1599) -> ()  [unwired: 2 in, 2 out]
        n1746 = property on="Home" class="Bool (strict)"("DisabledEnum"=w1599) -> ()  [unwired: 2 in, 2 out]
        n1747 = property on="Report" class="Bool (strict)"("DisabledEnum"=w1599) -> ()  [unwired: 2 in, 2 out]
      }
    }
    n1748 = local read "Quit"() -> (w1527:bool)
    "Single" <- "Single - Graph"
  }
  n1749 = disable-structure shown="Disabled" {
    disable-tunnel: [w1880 _] -> w46
    disable-tunnel: _ -> [w1879 _]
    frame Disabled {
      n1750 = while {
        tunnel: w1879 -> [_]
        tunnel: [w1881] -> w1880
        tunnel: [w1882] -> _
        i -> [w1882]
        stop <- w1881 stop-if-true
        w1898 = u16 10 items=["1.0"=10, "1.5"=15, "2.0"=20] ("stop bits (10: 1 bit)")
        n1751 = Wait (ms)(milliseconds to wait=u32 10) -> ()  [unwired: 1 out]
        n1752 = call-poly "VISA Configure Serial Port"("VISA resource name"=refnum<visa-resource-name> "ASRL1::INSTR" ("COM PORT"), "timeout (10sec)"=u32 10, "baud rate (9600)"=u32 57600, "data bits (8)"=u16 8, "stop bits (10: 1 bit)"=w1898) -> ("VISA resource name out"=w1884:refnum<visa-resource-name>, "error out"=w1893:errorcluster)  [unwired: 9 in]
        n1753 = VISA Read(VISA resource name=w1884, byte count=u32 2 ("byte count (0)")) -> (read buffer=w1892:string)  [unwired: 1 in, 3 out]
        n1754 = String Subset(string=w1892, offset (0)=0, length (rest)=2 ("length (rest)")) -> (substring=w1891:string)
        n1755 = Match Pattern(string=w1891, regular expression="<>") -> (offset past match=w1888:i32)  [unwired: 1 in, 3 out]
        n1756 = Greater Or Equal?(x=w1888, y=0) -> (x >= y?=w1883:bool)
        n1757 = case shown="True" w1883 {
          tunnel: w1884 -> [_ w1902]
          tunnel: w1893 -> [_ w1901]
          frame False {
          }
          frame True {
            n1758 = VISA Read(VISA resource name=w1902, byte count=u32 32 ("byte count (0)"), error in (no error)=w1901) -> (read buffer=w1900:string)  [unwired: 3 out]
            n1759 = String Subset(string=w1900, offset (0)=0, length (rest)=8 ("length (rest)")) -> (substring=w1904:string)
            n1760 = String Subset(string=w1900, offset (0)=8, length (rest)=8 ("length (rest)")) -> (substring=w1905:string)
            n1761 = Decimal String To Number(string=w1905) -> (number=w1912:i32)  [unwired: 2 in, 1 out]
            n1762 = Decimal String To Number(string=w1904) -> (number=w1908:i32)  [unwired: 2 in, 1 out]
            n1763 = Divide(x=w1912, y=10000) -> ()  [unwired: 1 out]
            n1764 = Divide(x=w1908, y=1000000) -> ()  [unwired: 1 out]
          }
        }
        n1765 = local read "Quit"() -> (w1881:bool)
      }
    }
    frame Enabled {
    }
  }
  n1766 = Tick Count (ms)() -> (millisecond timer value=w8:u32)
  n1767 = while {
    shift-right: [w1958] -> _
    shift-left: w10 -> [w1962]
    shift-right: [w1957] -> _
    shift-left: w9 -> [w1961]
    shift-right: [w1956] -> _
    shift-left: w10 -> [w1960]
    shift-right: [w1955] -> _
    shift-left: w9 -> [w1959]
    shift-right: [w1953] -> _
    shift-left: w8 -> [w1954]
    shift-right: [w1950] -> _
    shift-left: w7 -> [w1951]
    shift-right: [w1949] -> _
    shift-left: w7 -> [w1952]
    shift-right: [w1942] -> _
    shift-left: w7 -> [w1948]
    shift-right: [w1941] -> _
    shift-left: w7 -> [w1947]
    shift-right: [w1940] -> _
    shift-left: w7 -> [w1946]
    shift-right: [w1939] -> _
    shift-left: w7 -> [w1945]
    shift-right: [w1938] -> _
    shift-left: w7 -> [w1944]
    shift-right: [w1937] -> _
    shift-left: w7 -> [w1943]
    shift-right: [w1936] -> _
    shift-left: w7 -> [w1930]
    shift-right: [w1935] -> _
    shift-left: w7 -> [w1929]
    shift-right: [w1934] -> _
    shift-left: w7 -> [w1928]
    shift-right: [w1933] -> _
    shift-left: w7 -> [w1927]
    shift-right: [w1932] -> _
    shift-left: w7 -> [w1926]
    shift-right: [w1931] -> _
    shift-left: w7 -> [w1925]
    shift-right: [w1916] -> _
    shift-left: w7 -> [w1919]
    shift-right: [w1915] -> _
    shift-left: w7 -> [w1918]
    shift-right: [w1914] -> _
    shift-left: w7 -> [w1917]
    stop <- w1964 stop-if-true
    n1768 = local read "Read UNO"() -> (w1923:string)
    n1769 = local read "Error  2"() -> (w1963:errorcluster)
    n1770 = String Length(string=w1923) -> (length=w1922:i32)
    n1771 = call <vilib>:"Trim Whitespace.vi"("string"=w1923) -> ("trimmed string"=w1924:string)  [unwired: 1 in]
    n1772 = Greater Or Equal?(x=w1922, y=23) -> (x >= y?=w1920:bool)
    n1773 = case shown="No Error" w1963 {
      tunnel: w1962 -> [w2010 w2106]
      tunnel: w1961 -> [w2009 w2105]
      tunnel: w1960 -> [w2008 w2104]
      tunnel: w1959 -> [w2007 w2103]
      tunnel: [w2006 w2106] -> w1958
      tunnel: [w2005 w2105] -> w1957
      tunnel: [w2004 w2104] -> w1956
      tunnel: [w2003 w2103] -> w1955
      tunnel: w1954 -> [w2002 w2102]
      tunnel: [w2001 w2102] -> w1953
      tunnel: w1951 -> [w2000 w2101]
      tunnel: w1952 -> [w1999 w2100]
      tunnel: [w1998 w2101] -> w1950
      tunnel: [w1997 w2100] -> w1949
      tunnel: w1948 -> [w1996 w2099]
      tunnel: w1947 -> [w1995 w2098]
      tunnel: w1946 -> [w1994 w2097]
      tunnel: w1945 -> [w1993 w2096]
      tunnel: w1944 -> [w1992 w2095]
      tunnel: w1943 -> [w1991 w2094]
      tunnel: [w1990 w2099] -> w1942
      tunnel: [w1989 w2098] -> w1941
      tunnel: [w1988 w2097] -> w1940
      tunnel: [w1987 w2096] -> w1939
      tunnel: [w1986 w2095] -> w1938
      tunnel: [w1985 w2094] -> w1937
      tunnel: w1930 -> [w1984 w2093]
      tunnel: [w1983 w2093] -> w1936
      tunnel: [w1982 w2089] -> w1935
      tunnel: [w1981 w2088] -> w1934
      tunnel: [w1980 w2092] -> w1933
      tunnel: [w1979 w2091] -> w1932
      tunnel: [w1978 w2090] -> w1931
      tunnel: w1929 -> [w1977 w2092]
      tunnel: w1928 -> [w1976 w2091]
      tunnel: w1927 -> [w1975 w2090]
      tunnel: w1926 -> [w1974 w2089]
      tunnel: w1925 -> [w1973 w2088]
      tunnel: w1924 -> [w1972 _]
      tunnel: w1920 -> [w1971 _]
      tunnel: w1919 -> [w1970 w2087]
      tunnel: w1918 -> [w1969 w2086]
      tunnel: w1917 -> [w1968 w2085]
      tunnel: [w1967 w2087] -> w1916
      tunnel: [w1966 w2086] -> w1915
      tunnel: [w1965 w2085] -> w1914
      frame No Error {
        n1774 = case shown="True" w1971 {
          tunnel: w2010 -> [w2026 w2078]
          tunnel: w2009 -> [w2025 w2077]
          tunnel: w2008 -> [w2024 w2076]
          tunnel: w2007 -> [w2023 w2075]
          tunnel: [w2026 w2074] -> w2006
          tunnel: [w2025 w2073] -> w2005
          tunnel: [w2024 w2072] -> w2004
          tunnel: [w2023 w2071] -> w2003
          tunnel: w2002 -> [w2022 w2069]
          tunnel: [w2022 w2068] -> w2001
          tunnel: w2000 -> [w2021 w2067]
          tunnel: w1999 -> [w2020 w2066]
          tunnel: [w2021 w2065] -> w1998
          tunnel: [w2020 w2064] -> w1997
          tunnel: w1996 -> [w2019 w2063]
          tunnel: w1995 -> [w2018 w2062]
          tunnel: w1994 -> [w2017 w2061]
          tunnel: w1993 -> [w2016 w2060]
          tunnel: w1992 -> [w2015 w2059]
          tunnel: w1991 -> [w2014 w2058]
          tunnel: [w2019 w2057] -> w1990
          tunnel: [w2018 w2056] -> w1989
          tunnel: [w2017 w2055] -> w1988
          tunnel: [w2016 w2054] -> w1987
          tunnel: [w2015 w2053] -> w1986
          tunnel: [w2014 w2052] -> w1985
          tunnel: w1984 -> [w2032 w2051]
          tunnel: [w2032 w2050] -> w1983
          tunnel: [w2029 w2049] -> w1982
          tunnel: [w2028 w2048] -> w1981
          tunnel: [w2031 w2047] -> w1980
          tunnel: [w2027 w2046] -> w1979
          tunnel: [w2030 w2045] -> w1978
          tunnel: w1977 -> [w2031 w2044]
          tunnel: w1976 -> [w2030 w2043]
          tunnel: w1975 -> [w2029 w2042]
          tunnel: w1974 -> [w2028 w2041]
          tunnel: w1973 -> [w2027 w2040]
          tunnel: w1972 -> [_ w2039]
          tunnel: w1970 -> [w2013 w2038]
          tunnel: w1969 -> [w2012 w2037]
          tunnel: w1968 -> [w2011 w2036]
          tunnel: [w2013 w2035] -> w1967
          tunnel: [w2012 w2034] -> w1966
          tunnel: [w2011 w2033] -> w1965
          frame False {
          }
          frame True {
            n1775 = Tick Count (ms)() -> (millisecond timer value=w2070:u32)
            n1776 = String To Byte Array(string=w2039) -> (unsigned byte array=w2083:u8[])
            n1777 = Array Size(array=w2083) -> (size(s)=w2082:i32)
            n1778 = formula code="// --- INTERNAL VARIABLE DECLARATIONS ---\nint i = 0;\nint k = 0;\nint start_idx = -1;\nint end_idx = -1;\nint phase = 0;\nint sign0 = 1;\nint sign1 = 1;\nint ch0_val = 0;   \nint ch1_val = 0;   \nfloat ch0_raw = 0.0;\nfloat ch1_raw = 0.0;\nfloat temp0 = 0.0;\nfloat temp1 = 0.0;\nfloat ch0_clean = 0.0;\nfloat ch1_clean = 0.0;\n\nint valid_samples = 0; // FIX: Track if we actually parsed new data this window\nfloat max_allowed_bits = 8388607.0; // FIX: Change this to match your ADC max value\n\n// Temporal intermediate variables for calculation smoothing\nfloat raw_p2p_v = 0.0;\nfloat raw_friction = 0.0;\nfloat raw_cof = 0.0;\n\n// Temporal intermediate variables for Piezo voltage translations\nfloat piezo_min_v = 0.0;\nfloat piezo_max_v = 0.0;\n\n// Initialize output variables to current shift register states right away\nout_LVDT_Min_V = in_LVDT_Min_V;\nout_LVDT_Max_V = in_LVDT_Max_V;\nout_LVDT_P2P_V = in_LVDT_P2P_V;\nout_Piezo_P2P = in_Piezo_P2P;\nout_Friction_N = in_Friction_N;\nout_COF = in_COF;\nwindow_ready = 0;\n\n// --- STEP 1: PARSE EVERY STRING IN THE BYTE ARRAY ---\nif (array_size > 2) {\n    for (i = 0; i < array_size - 1; i++) {\n        if (raw_bytes[i] == 42) { // '*' character detected\n            start_idx = i;\n        }\n        \n        // Match standard delimiter sequence \";&\" or end window character\n        if (raw_bytes[i] == 59 && raw_bytes[i+1] == 38 && start_idx != -1) { \n            end_idx = i;\n            ch0_val = 0;\n            ch1_val = 0;\n            sign0 = 1;\n            sign1 = 1;\n            phase = 0; \n\n            for (k = start_idx + 1; k < end_idx; k++) {\n                if (raw_bytes[k] == 45) { // '-' sign\n                    if (phase == 0) sign0 = -1;\n                    else sign1 = -1;\n                }\n                else if (raw_bytes[k] == 43) { // '+' sign\n                    if (phase == 0) sign0 = 1;\n                    else sign1 = 1;\n                }\n                else if (raw_bytes[k] == 59) { // ';' delimiter\n                    phase = 1; \n                }\n                else if (raw_bytes[k] >= 48 && raw_bytes[k] <= 57) { // Numeric ASCII digits\n                    if (phase == 0) {\n                        ch0_val = (ch0_val * 10) + (raw_bytes[k] - 48);\n                    } else {\n                        ch1_val = (ch1_val * 10) + (raw_bytes[k] - 48);\n                    }\n                }\n            }\n\n            // Implicit type conversion\n            ch0_raw = ch0_val * sign0 * 1.0;\n            ch1_raw = ch1_val * sign1 * 1.0;\n\n            // FIX: Sanity check / Hard-clamping to catch sudden massive ASCII noise spikes\n            if (ch0_raw > max_allowed_bits)  ch0_raw = max_allowed_bits;\n            if (ch0_raw < -max_allowed_bits) ch0_raw = -max_allowed_bits;\n            if (ch1_raw > max_allowed_bits)  ch1_raw = max_allowed_bits;\n            if (ch1_raw < -max_allowed_bits) ch1_raw = -max_allowed_bits;\n\n            // --- STEP 2: 3-SAMPLE MEDIAN FILTER ---\n            m0_2 = m0_1; m0_1 = m0_0; m0_0 = ch0_raw;\n            float s0_0 = m0_0; float s0_1 = m0_1; float s0_2 = m0_2;\n            if (s0_0 > s0_1) { temp0 = s0_0; s0_0 = s0_1; s0_1 = temp0; }\n            if (s0_1 > s0_2) { temp0 = s0_1; s0_1 = s0_2; s0_2 = temp0; }\n            if (s0_0 > s0_1) { temp0 = s0_0; s0_0 = s0_1; s0_1 = temp0; }\n            ch0_clean = s0_1;\n\n            m1_2 = m1_1; m1_1 = m1_0; m1_0 = ch1_raw;\n            float s1_0 = m1_0; float s1_1 = m1_1; float s1_2 = m1_2;\n            if (s1_0 > s1_1) { temp1 = s1_0; s1_0 = s1_1; s1_1 = temp1; }\n            if (s1_1 > s1_2) { temp1 = s1_1; s1_1 = s1_2; s1_2 = temp1; }\n            if (s1_0 > s1_1) { temp1 = s1_0; s1_0 = s1_1; s1_1 = temp1; }\n            ch1_clean = s1_1;\n\n            // --- STEP 3: EXPONENTIAL FILTER (STREAM LEVEL) ---\n            if (ch0_filt == 0.0) ch0_filt = ch0_clean;\n            if (ch1_filt == 0.0) ch1_filt = ch1_clean;\n\n            ch0_filt = ch0_filt + (ch0_clean - ch0_filt) * 0.125;\n            ch1_filt = ch1_filt + (ch1_clean - ch1_filt) * 0.125;\n\n            // --- STEP 4: MIN/MAX WINDOW CONTINUOUS ACCUMULATION ---\n            if (ch0_filt > max_ch0) max_ch0 = ch0_filt;\n            if (ch0_filt < min_ch0) min_ch0 = ch0_filt;\n            if (ch1_filt > max_ch1) max_ch1 = ch1_filt;\n            if (ch1_filt < min_ch1) min_ch1 = ch1_filt;\n\n            valid_samples++; // FIX: Successfully parsed and accumulated a clean point\n            start_idx = -1; \n        }\n    }\n}\n\n// --- STEP 5: WINDOW EVALUATION ENGINE ---\n// FIX: Condition updated to verify that valid samples exist for both channels\nif (((current_time_ms - start_time_ms) >= 50) && (valid_samples > 0) && (min_ch0 < 9000000.0) && (min_ch1 < 9000000.0)) {\n    window_ready = 1;\n\n    // Linear Bit-to-Voltage Transformations (LVDT - Channel 0)\n    out_LVDT_Min_V = (min_ch0 * VREF) / 8388607.0;\n    out_LVDT_Max_V = (max_ch0 * VREF) / 8388607.0;\n    raw_p2p_v = out_LVDT_Max_V - out_LVDT_Min_V;\n\n    // Linear Bit-to-Voltage Transformations (Piezo - Channel 1)\n    piezo_min_v = (min_ch1 * VREF) / 8388607.0;\n    piezo_max_v = (max_ch1 * VREF) / 8388607.0;\n    \n    // Assign Peak-to-Peak Voltage directly to output indicator (Matches Python logic)\n    out_Piezo_P2P = piezo_max_v - piezo_min_v;\n    \n    // Force scaling calculations using Voltage delta * Newtons/Volt Factor\n    raw_friction = out_Piezo_P2P * PIEZO_CAL_FACTOR ;\n    raw_cof = raw_friction / NORMAL_FORCE;\n\n    // --- STEP 6: OUTPUT METRIC SMOOTHING (Low-Pass Filter Alpha = 0.05) ---\n    // Seed initial historical metrics if first loop iteration\n    if (hist_LVDT_P2P == 0.0) hist_LVDT_P2P = raw_p2p_v;\n    if (hist_Friction == 0.0) hist_Friction = raw_friction;\n    if (hist_COF == 0.0)      hist_COF = raw_cof;\n\n    // Apply exponential output dampening\n    hist_LVDT_P2P = hist_LVDT_P2P + (raw_p2p_v - hist_LVDT_P2P) * 0.05;\n    hist_Friction = hist_Friction + (raw_friction - hist_Friction) * 0.05; // Note: Can drop to 0.02 for more aggressive damping\n    hist_COF      = hist_COF + (raw_cof - hist_COF) * 0.05;\n\n    // Direct smoothed parameters out to UI Indicators\n    out_LVDT_P2P_V = hist_LVDT_P2P;\n    out_Friction_N = hist_Friction;\n    out_COF        = hist_COF;\n\n    // Reset tracking targets to extreme boundaries safely\n    min_ch0 = 9999999.0;\n    max_ch0 = -9999999.0;\n    min_ch1 = 9999999.0;\n    max_ch1 = -9999999.0;\n\n    valid_samples = 0; // FIX: Reset counter for next time frame\n    start_time_ms = current_time_ms;\n}"("raw_bytes"=w2083, "array_size"=w2082, "VREF"="VREF", "PIEZO_CAL_FACTOR"="PIEZO_CAL_FACTOR", "NORMAL_FORCE"="NORMAL_FORCE", "min_ch0"=w2078, "max_ch0"=w2077, "min_ch1"=w2076, "max_ch1"=w2075, "current_time_ms"=w2070, "start_time_ms"=w2069, "ch0_filt"=w2067, "ch1_filt"=w2066, "m0_0"=w2063, "m0_1"=w2062, "m0_2"=w2061, "m1_0"=w2060, "m1_1"=w2059, "m1_2"=w2058, "in_LVDT_Min_V"=w2051, "in_LVDT_Max_V"=w2044, "in_LVDT_P2P_V"=w2043, "in_Piezo_P2P"=w2042, "in_Friction_N"=w2041, "in_COF"=w2040, "hist_LVDT_P2P"=w2038, "hist_Friction"=w2037, "hist_COF"=w2036) -> ("window_ready"=→"Valid_data":dbl, "out_LVDT_Min_V"=w2050:dbl, "out_LVDT_Max_V"=w2049:dbl, "out_LVDT_P2P_V"=w2048:dbl, "out_Piezo_P2P"=w2047:dbl, "out_Friction_N"=w2046:dbl, "out_COF"=w2045:dbl, "min_ch0"=w2074:dbl, "max_ch0"=w2073:dbl, "min_ch1"=w2072:dbl, "max_ch1"=w2071:dbl, "start_time_ms"=w2068:u32, "ch0_filt"=w2065:dbl, "ch1_filt"=w2064:dbl, "m0_0"=w2057:dbl, "m0_1"=w2056:dbl, "m0_2"=w2055:dbl, "m1_0"=w2054:dbl, "m1_1"=w2053:dbl, "m1_2"=w2052:dbl, "hist_LVDT_P2P"=w2035:dbl, "hist_Friction"=w2034:dbl, "hist_COF"=w2033:dbl)